vi "HFRR ADV v043.vi"() -> ()   [LabVIEW 2025] (continued)
            "LVDT MIN" <- w2050
            "LVDT MAX" <- w2049
            "LVDT Peak" <- w2048
            "pizo raw" <- w2047
            "cof" <- w2045
            "Frictioin Force Raw" <- w2046
          }
        }
      }
      frame Error {
      }
    }
    n1779 = local read "Quit"() -> (w1964:bool)
  }
  n1780 = disable-structure shown="Disabled" {
    disable-tunnel: errorcluster {"status"=TRUE, "code"=0, "source"="Init"} ("error IO") -> [w2109 _]
    disable-tunnel: [w2107 _] -> w49
    frame Disabled {
      n1781 = while {
        shift-right: [w2125] -> w2111
        shift-left: _ -> [w2116]
        shift-right: [w2124] -> w2110
        shift-left: w2109 -> [w2118]
        tunnel: [w2113] -> w2107
        tunnel: [w2123] -> _
        i -> [w2123]
        stop <- w2113 stop-if-true
        n1782 = local read "Port 1a"() -> (w2119:bool)
        n1783 = local read "Port 3"() -> (w2120:bool)
        n1784 = local read "Com Port 1"() -> (w2117:refnum<visa-resource-name>)
        n1785 = Or(x=w2120, y=w2119) -> (x .or. y?=w2122:bool)
        n1786 = Unbundle(w2118) -> ("status"=→"Port 3":bool)  [unwired: 2 out]
        n1787 = Not Equal?(x=w2117, y=w2116) -> (x != y?=w2114:bool)
        n1788 = case shown="True" w2122 {
          frame False {
            w2128 = TRUE ("Visible")
            n1789 = property on="Port 1a" class="Bool (strict)"("Visible"=w2128) -> ()  [unwired: 2 in, 2 out]
            n1790 = property on="Port 3" class="Bool (strict)"("Visible"=w2128) -> ()  [unwired: 2 in, 2 out]
          }
          frame True {
            w2129 = TRUE ("Visible")
            n1791 = property on="Port 1a" class="Bool (strict)"("Visible"=w2129) -> ()  [unwired: 2 in, 2 out]
            n1792 = property on="Port 3" class="Bool (strict)"("Visible"=w2129) -> ()  [unwired: 2 in, 2 out]
          }
        }
        n1793 = Wait (ms)(milliseconds to wait=u32 40) -> ()  [unwired: 1 out]
        n1794 = case shown="True" w2114 {
          tunnel: [w2126 errorcluster {"status"=TRUE, "code"=0, "source"="Init"} ("error out")] -> w2115
          tunnel: w2118 -> [w2126 _]
          frame False {
          }
          frame True {
          }
        }
        n1795 = case shown="Error" w2115 {
          selector: w2115 -> [w2136 w2154]
          tunnel: [w2139 w2158] -> w2125
          tunnel: [w2138 w2152] -> w2124
          tunnel: w2116 -> [w2137 w2156]
          frame No Error {
            n1796 = property class="Instr"(reference=w2137, error in=w2136) -> (reference out=w2134:refnum<visa-resource-name>, error out=w2135:errorcluster, "Serial Settings:Number of Bytes at Serial Port"=w2131:u32)
            n1797 = Greater?(x=w2131, y=u32 5) -> (0:w2130:bool)
            n1798 = Not(x=w2130) -> (.not. x?=→"Port 1a":bool)
            n1799 = while {
              tunnel: [w2147] -> w2138
              tunnel: [w2146] -> w2139
              tunnel: w2135 -> [w2145]
              tunnel: w2134 -> [w2144]
              stop <- TRUE stop-if-true
              n1800 = property class="Instr" props=["Serial Settings:Number of Bytes at Serial Port"](reference=w2144, error in=w2145) -> (reference out=w2149:refnum<visa-resource-name>, error out=w2148:errorcluster)  [unwired: 1 out]
              n1801 = VISA Read(VISA resource name=w2149, byte count=u32 50, error in (no error)=w2148) -> (VISA resource name out=w2146:refnum<visa-resource-name>, read buffer=w2141:string, error out=w2147:errorcluster)  [unwired: 1 out]
              n1802 = Wait (ms)(milliseconds to wait=u32 5) -> ()  [unwired: 1 out]
            }
          }
          frame Error {
            w2164 = u16 0 items=["None", "XON/XOFF", "RTS/CTS", "XON/XOFF & RTS/CTS", "DTR/DSR", "XON/XOFF & DTR/DSR"] ("flow control (0:none)  2")
            w2162 = u16 10 items=["1.0"=10, "1.5"=15, "2.0"=20] ("stop bits 2")
            w2160 = u16 0 items=["None", "Odd", "Even", "Mark", "Space"] ("parity 2")
            w2161 = u32 10000  # timeout (10sec)
            n1803 = VISA Close(VISA resource name=w2156, error in (no error)=w2154) -> (error out=w2157:errorcluster)
            n1804 = local write "Port 1a"(FALSE ("Port 1a")) -> ()
            n1805 = local read "Com Port 1"() -> (w2151:refnum<visa-resource-name>)
            n1806 = call <vilib>:"Clear Errors.vi"("error in (no error)"=w2157) -> ("error out"=w2155:errorcluster)  [unwired: 5 in, 1 out]
            n1807 = call-poly "VISA Configure Serial Port"("VISA resource name"=w2151, "timeout (10sec)"=w2161, "baud rate (9600)"=u32 250000 ("baud rate  2"), "data bits (8)"=u16 8 ("data bits  2"), "parity (0:none)"=w2160, "error in (no error)"=w2155, "stop bits (10: 1 bit)"=w2162, "flow control (0:none)"=w2164) -> ("VISA resource name out"=w2165:refnum<visa-resource-name>, "error out"=w2166:errorcluster)  [unwired: 6 in]
            n1808 = flat-sequence {
              tunnel: w2165 -> [w2168]
              tunnel: w2166 -> [w2167]
              tunnel: [w2168] -> w2158
              tunnel: [w2167] -> w2152
              frame #0 {
                n1809 = Wait (ms)(milliseconds to wait=u32 50) -> ()  [unwired: 1 out]
              }
            }
            "Residual Uno" <- ""
          }
        }
        n1810 = local read "Quit"() -> (w2113:bool)
        "Error Uno" <- w2118
      }
      n1811 = VISA Close(VISA resource name=w2111, error in (no error)=w2110) -> (error out=w2108:errorcluster)
      n1812 = call <vilib>:"Clear Errors.vi"("error in (no error)"=w2108) -> ()  [unwired: 5 in, 2 out]
    }
    frame Enabled {
    }
  }
  n1813 = while {
    stop <- w2179 stop-if-true
    # "V0OLTAGE TO STROKE (peice vise calibration)"
    n1814 = local read "LVDT MIN"() -> (w2171:dbl)
    n1815 = local read "LVDT Peak"() -> (w2170:dbl)
    n1816 = Wait (ms)(milliseconds to wait=u32 10) -> ()  [unwired: 1 out]
    n1817 = formula code="// Dynamic Parameterized Linear Interpolation Node\n// Inputs: vpp_val, voltages (Array), distances (Array)\n// Outputs: stroke\n\nint i = 0;\nint segments = 11; // 12 points make 11 interpolation segments\n\n// 1. Lower Boundary Clamp\nif (vpp_val <= voltages[0]) {\n    stroke = distances[0];\n}\n// 2. Upper Boundary Clamp\nelse if (vpp_val >= voltages[segments]) {\n    stroke = distances[segments];\n}\n// 3. Dynamic Segment Search Loop\nelse {\n    stroke = distances[0]; // Fallback baseline\n    for (i = 0; i < segments; i++) {\n        if (vpp_val >= voltages[i] && vpp_val <= voltages[i+1]) {\n            // Standard linear interpolation formula using array lookups\n            stroke = distances[i] + (vpp_val - voltages[i]) * (distances[i+1] - distances[i]) / (voltages[i+1] - voltages[i]);\n            break; // Segment found, safely exit the loop\n        }\n    }\n}"("vpp_val"=w2170, "voltages"="calibration values", "distances"="STROKE") -> ("stroke"=→"LVDT STROKE":dbl)
    n1818 = local read "Calibration Tare Value"() -> (w2175:dbl)
    n1819 = local read "Calibration Tare"() -> (w2173:bool)
    n1820 = Subtract(x=w2171, y=w2175) -> (x-y=→"LVDT STROKE  Calibration":dbl)
    n1821 = case shown="True" w2173 {
      selector: w2173 -> [_ w2181]
      tunnel: w2171 -> [_ w2182]
      frame False {
      }
      frame True {
        n1822 = Not(x=w2181) -> (.not. x?=w2180:bool)
        n1823 = local write "Calibration Tare"(w2180) -> ()
        "Calibration Tare Value" <- w2182
      }
    }
    n1824 = local read "Quit"() -> (w2179:bool)
  }
  n1825 = while {
    stop <- w2205 stop-if-true
    n1826 = local read "Due read"() -> (w2203:string)
    n1827 = call <vilib>:"High Resolution Polling Wait.vi"("seconds to wait"=0.02) -> ()  [unwired: 10 in, 1 out]
    n1828 = local read "Frictioin Force Raw"() -> (w2185:dbl)
    n1829 = Spreadsheet String To Array(delimiter (Tab)=";", format string="", spreadsheet string=w2203, array type (2D Dbl)=string[] []) -> (array=w2200:string[])
    n1830 = Fract/Exp String To Number(string=w2200) -> (number=w2199:dbl[])  [unwired: 3 in, 1 out]
    n1831 = call <vilib>:"Median Filter PtByPt.vi"("rank"=2, "x"=w2185) -> ("Filtered x"=→"Friction":dbl)  [unwired: 2 in, 1 out]
    n1832 = Index Array(array=w2199) -> (element #1=→"Sample Temperature 2":dbl, element #2=→"Target Sample Temperature":dbl, element #3=→"Current Duty Cycle":dbl, element #4=→"Ambient Temperature":dbl, element #5=→"Dac Status":dbl, element #6=→"Vpp":dbl, element #7=→"Active Error Code":dbl, element #8=→"Kp":dbl, element #9=→"Ki":dbl, element #10=→"Kd":dbl, element #11=→"SampleRaw":dbl, element #12=→"AmbRaw":dbl)  [unwired: 12 in]
    n1833 = local read "Quit"() -> (w2205:bool)
  }
  n1834 = while {
    shift-right: [w2219] -> w45
    shift-left: _ -> [w2211]
    shift-right: [w2206] -> w44
    shift-left: errorcluster {"status"=FALSE, "code"=0, "source"="Init"} ("error out") -> [w2213]
    tunnel: [w2208] -> w48
    tunnel: [w2218] -> _
    i -> [w2218]
    stop <- w2208 stop-if-true
    n1835 = local read "Com Port 2"() -> (w2212:refnum<visa-resource-name>)
    n1836 = local read "Port 2a"() -> (w2214:bool)
    n1837 = Unbundle(w2213) -> ("status"=→"Port 4":bool)  [unwired: 2 out]
    n1838 = call <vilib>:"High Resolution Polling Wait.vi"("seconds to wait"=0.02) -> ()  [unwired: 10 in, 1 out]
    n1839 = local read "Port 4"() -> (w2215:bool)
    n1840 = Not Equal?(x=w2212, y=w2211) -> (x != y?=w2210:bool)
    n1841 = Or(x=w2215, y=w2214) -> (x .or. y?=w2217:bool)
    n1842 = case shown="False" w2217 {
      frame False {
        w2222 = TRUE ("Visible")
        n1843 = property on="Port 2a" class="Bool (strict)"("Visible"=w2222) -> ()  [unwired: 2 in, 2 out]
        n1844 = property on="Port 4" class="Bool (strict)"("Visible"=w2222) -> ()  [unwired: 2 in, 2 out]
      }
      frame True {
        w2223 = TRUE ("Visible")
        n1845 = property on="Port 2a" class="Bool (strict)"("Visible"=w2223) -> ()  [unwired: 2 in, 2 out]
        n1846 = property on="Port 4" class="Bool (strict)"("Visible"=w2223) -> ()  [unwired: 2 in, 2 out]
      }
    }
    n1847 = case shown="True" w2210 {
      tunnel: [w2220 errorcluster {"status"=TRUE, "code"=0, "source"="Init"} ("error out")] -> w2209
      tunnel: w2213 -> [w2220 _]
      frame False {
      }
      frame True {
      }
    }
    n1848 = case shown="No Error" w2209 {
      selector: w2209 -> [w2236 w2267]
      tunnel: [w2229 w2272] -> w2219
      tunnel: [w2237 w2265] -> w2206
      tunnel: w2211 -> [w2238 w2270]
      frame No Error {
        n1849 = property class="Instr" props=["Serial Settings:Number of Bytes at Serial Port"](reference=w2238, error in=w2236) -> (reference out=w2230:refnum<visa-resource-name>, error out=w2235:errorcluster)  [unwired: 1 out]
        n1850 = while {
          tunnel: [w2246] -> w2231
          tunnel: [w2245] -> w2232
          tunnel: w2235 -> [w2244]
          tunnel: w2230 -> [w2243]
          tunnel: [w2242] -> _
          i -> [w2242]
          stop <- TRUE stop-if-true
          n1851 = property class="Instr" props=["Serial Settings:Number of Bytes at Serial Port"](reference=w2243, error in=w2244) -> (reference out=w2248:refnum<visa-resource-name>, error out=w2247:errorcluster)  [unwired: 1 out]
          n1852 = VISA Read(VISA resource name=w2248, byte count=u32 1000, error in (no error)=w2247) -> (VISA resource name out=w2245:refnum<visa-resource-name>, read buffer=→"Due read":string, error out=w2246:errorcluster)  [unwired: 1 out]
        }
        n1853 = local read "Due Write"() -> (w2228:string)
        n1854 = call <vilib>:"Trim Whitespace.vi"("string"=w2228) -> ("trimmed string"=w2227:string)  [unwired: 1 in]
        n1855 = Not Equal?(x=w2227, y="") -> (x != y?=w2233:bool)
        n1856 = VISA Flush I/O Buffer(VISA resource name=w2232) -> (VISA resource name out=w2225:refnum<visa-resource-name>, error out=→"error out 10":errorcluster)  [unwired: 2 in]
        n1857 = case shown="True" w2233 {
          tunnel: w2225 -> [w2250 w2255]
          tunnel: [w2250 w2259] -> w2229
          tunnel: w2231 -> [w2249 w2254]
          tunnel: [w2249 w2257] -> w2237
          tunnel: w2227 -> [_ w2253]
          tunnel: [_ w2256] -> _
          frame False {
            # "DATA  WRITE LOOP"
          }
          frame True {
            n1858 = Concatenate Strings(w2253, "\r\n") -> (w2252:string)
            n1859 = VISA Write(VISA resource name=w2255, write buffer=w2252, error in (no error)=w2254) -> (VISA resource name out=w2259:refnum<visa-resource-name>, return count=w2256:u32, error out=w2258:errorcluster)
            n1860 = flat-sequence {
              tunnel: w2258 -> [w2261]
              tunnel: [w2261] -> w2257
              frame #0 {
                n1861 = local write "Due Write"("" ("Command")) -> ()
                n1862 = Wait (ms)(milliseconds to wait=u32 5) -> ()  [unwired: 1 out]
              }
            }
          }
        }
        "Port 2a" <- TRUE ("Port 2a")
      }
      frame Error {
        w2278 = u16 0 items=["None", "XON/XOFF", "RTS/CTS", "XON/XOFF & RTS/CTS", "DTR/DSR", "XON/XOFF & DTR/DSR"] ("flow control (0:none)  2")
        w2276 = u16 10 items=["1.0"=10, "1.5"=15, "2.0"=20] ("stop bits 2")
        w2274 = u16 0 items=["None", "Odd", "Even", "Mark", "Space"] ("parity 2")
        w2275 = u32 10000  # timeout (10sec)
        n1863 = VISA Clear(VISA resource name=w2270, error in (no error)=w2267) -> (VISA resource name out=w2269:refnum<visa-resource-name>, error out=w2268:errorcluster)
        n1864 = VISA Close(VISA resource name=w2269, error in (no error)=w2268) -> (error out=w2271:errorcluster)
        n1865 = call <vilib>:"Clear Errors.vi"("error in (no error)"=w2271) -> ()  [unwired: 5 in, 2 out]
        n1866 = local write "Port 2a"(FALSE ("Port 2a")) -> ()
        n1867 = local read "Com Port 2"() -> (w2264:refnum<visa-resource-name>)
        "visa due" <- w2264
        n1868 = call-poly "VISA Configure Serial Port"("VISA resource name"=w2264, "timeout (10sec)"=w2275, "baud rate (9600)"=u32 250000 ("baud rate  2"), "data bits (8)"=u16 8 ("data bits  2"), "parity (0:none)"=w2274, "stop bits (10: 1 bit)"=w2276, "flow control (0:none)"=w2278) -> ("VISA resource name out"=w2279:refnum<visa-resource-name>, "error out"=w2280:errorcluster)  [unwired: 7 in]
        n1869 = flat-sequence {
          tunnel: w2279 -> [w2282]
          tunnel: w2280 -> [w2281]
          tunnel: [w2282] -> w2272
          tunnel: [w2281] -> w2265
          frame #0 {
            n1870 = Wait (ms)(milliseconds to wait=u32 50) -> ()  [unwired: 1 out]
          }
        }
        "Residual Due" <- ""
      }
    }
    "error out 9" <- w2206
    n1871 = local read "Quit"() -> (w2208:bool)
    "Error Due" <- w2213
  }
  n1872 = local write "FRICVALZ"(0.0 ("FRICVALZ")) -> ()
  n1873 = property on="RUN" class="Bool (strict)"("Visible"=TRUE) -> ()  [unwired: 2 in, 2 out]
  n1874 = while {
    tunnel: [w2297] -> _
    tunnel: [w2284] -> w58
    i -> [w2297]
    stop <- w2284 stop-if-true
    n1875 = local read "conststatus"() -> (w2288:dbl)
    n1876 = local read "Main Tab"() -> (w2286:T2)
    n1877 = local read "EDIT"() -> (w2303:bool)
    n1878 = local read "Rate"() -> (w2302:dbl)
    n1879 = case shown="True" w2303 {
      tunnel: [FALSE TRUE] -> _
      frame False {
      }
      frame True {
      }
    }
    n1880 = Equal?(x=w2286, y=T28."About" ("Main Tab")) -> (x = y?=w2295:bool)
    n1881 = Equal?(x=w2288, y=0.0) -> (x = y?=w2289:bool)
    n1882 = Divide(x=1.0, y=w2302) -> (x/y=w2298:dbl)
    "Time 2" <- w2298
    n1883 = case shown="True" w2289 {
      frame False {
      }
      frame True {
        # "C:\\WinDucom\\calibrate WO 2391.dcf"
        n1884 = local write "Lan flag"(22) -> ()
        n1885 = local write "conststatus"(10.0 ("rpm value : 2")) -> ()
        n1886 = String To Path(string="C:\\LAB-IQ\\calibrate WO 2465.dcf") -> (path=w2309:path)
        n1887 = Open/Create/Replace File "Open File"(file path (use dialog)=w2309) -> (refnum out=w2307:refnum<file>)  [unwired: 5 in, 2 out]
        n1888 = for {
          N: 23 -> [_]
          tunnel: w2307 -> [w2318]
          i -> [w2312]
          (unwired) TRUE ("line mode (F)")
          n1889 = Read from Text File "Read File"(file (use dialog)=w2318) -> (text=w2317:string)  [unwired: 3 in, 3 out]
          n1890 = Match Pattern(string=w2317, regular expression="]") -> (after substring=w2315:string)  [unwired: 1 in, 3 out]
          n1891 = String Subset(string=w2317, offset (0)=5, length (rest)=10 ("length (rest)")) -> (substring=w2310:string)
          n1892 = Fract/Exp String To Number(string=w2310) -> (number=w2311:dbl)  [unwired: 3 in, 1 out]
          n1893 = Match Pattern(string=w2315, regular expression="-") -> (before substring=w2313:string)  [unwired: 1 in, 3 out]
          n1894 = case shown="10" w2312 {
            tunnel: w2311 -> [_ _ _ _ _ _ _ _ _ _ w2325 _ _ _ _ _ _ _ _ _ _ _ _ _]
            tunnel: w2313 -> [_ _ _ _ w2321 w2322 w2323 _ _ _ _ _ _ _ _ _ _ _ _ _ w2326 w2327 w2328 _]
            frame 0 {
            }
            frame 1 {
            }
            frame 2 {
            }
            frame 3 {
            }
            frame 4 {
              n1895 = local write "Com Port 1"(w2321) -> ()
            }
            frame 5 {
              n1896 = local write "Com Port 2"(w2322) -> ()
              n1897 = local write "visa due"(w2322) -> ()
            }
            frame 6 {
              n1898 = String To Path(string=w2323) -> (path=w2324:path)
              n1899 = local write "File Path"(w2324) -> ()
              "String" <- w2323
            }
            frame 7 {
            }
            frame 8 {
            }
            frame 9 {
            }
            frame 10 {
              n1900 = local write "Language Selection"(w2325) -> ()
            }
            frame 11 {
            }
            frame 12 {
            }
            frame 13 {
            }
            frame 14 {
            }
            frame 15 {
            }
            frame 16 {
            }
            frame 17 {
            }
            frame 18 {
            }
            frame 21 {
            }
            frame 22 {
              n1901 = local write "Com Port 3"(w2326) -> ()
            }
            frame 20 {
              n1902 = local write "Camera Port :"(w2327) -> ()
            }
            frame 19 {
              n1903 = local write "C3 :"(w2328) -> ()
            }
            frame 23, Default {
            }
          }
        }
      }
    }
    n1904 = Select(t=u32 2500 ("milliseconds to wait"), s=w2295, f=u32 500 ("milliseconds to wait")) -> (s? t:f=w2293:u32)
    n1905 = Multiply(x=w2298, y=w2293) -> (x*y=w2300:dbl)
    n1906 = call "Elapsed Time2"("Time Target (s)"=w2300, "Auto Reset"=TRUE) -> ("Time has Elapsed"=w2290:bool)  [unwired: 10 in, 7 out]
    n1907 = case shown="True" w2290 {
      frame False {
      }
      frame True {
        n1908 = stacked-sequence {
          frame #0 {
            # "DATA PROCESSING"
            # "115 mV/N"
            n1909 = local read "Sample Temperature 2"() -> (w2331:dbl)
            n1910 = local read "RH Numeric:"() -> (→"Humidity ( %RH )":dbl)
            n1911 = local read "FRICVALZ"() -> (w2348:dbl)
            n1912 = local read "Friction"() -> (w2334:dbl)
            n1913 = call <vilib>:"Mean PtByPt.vi"("x"=w2331, "sample length"=100) -> ("mean"=w2330:dbl)  [unwired: 2 in, 1 out]
            "TEMP 2" <- w2330
            "TEMP 3" <- w2330
            n1914 = Subtract(x=w2334, y=w2348) -> (x-y=w2343:dbl)
            "FF 2" <- w2343
            "FF 4" <- w2343
            n1915 = local read "Ambient Temperature"() -> (→"AIR TEMP":dbl)
            n1916 = local read "TEMP"() -> (w2347:dbl)
            n1917 = local write "FF 3"(w2343) -> ()
            n1918 = Compound Arithmetic op=OR("FRICVALZ 4", "FRICVALZ 3", "FRICVALZ 2") -> (w2339:bool)
            n1919 = case shown="True" w2339 {
              tunnel: w2334 -> [_ w2354]
              frame False {
              }
              frame True {
                w2353 = FALSE ("FRICVALZ")
                n1920 = local write "FRICVALZ 3"(w2353) -> ()
                n1921 = local write "FRICVALZ 2"(w2353) -> ()
                n1922 = local write "FRICVALZ 4"(w2353) -> ()
                "FRICVALZ" <- w2354
              }
            }
            n1923 = Not A Number/Path/Refnum?(number/path/refnum=w2347) -> (NaN/Path/Refnum?=w2346:bool)
            n1924 = Not A Number/Path/Refnum?(number/path/refnum=w2343) -> (NaN/Path/Refnum?=w2345:bool)
            n1925 = Divide(x=w2343, y=1.96) -> (x/y=w2340:dbl)
            n1926 = Compound Arithmetic op=OR(w2346, w2345) -> (w2344:bool)
            n1927 = Not A Number/Path/Refnum?(number/path/refnum=w2340) -> (NaN/Path/Refnum?=w2341:bool)
            n1928 = case shown="True" w2344 {
              frame False {
              }
              frame True {
                n1929 = local write "TEMP"(0.0 ("TEMP")) -> ()
                n1930 = local write "FF 2"(0.0 ("FF 2")) -> ()
                n1931 = local write "reinit"(TRUE ("reinit")) -> ()
              }
            }
            n1932 = local write "TEMP"(w2330) -> ()
            n1933 = Select(t=0.0, s=w2341, f=w2340) -> (s? t:f=w2333:dbl)
            "COF 2" <- w2333
            n1934 = local write "COF 3"(w2333) -> ()
          }
        }
      }
    }
    n1935 = Wait (ms)(milliseconds to wait=u32 50) -> ()  [unwired: 1 out]
    n1936 = local read "Quit"() -> (w2284:bool)
    "Rate" <- 2500.0 ("No of Samples")
  }
  n1937 = while {
    tunnel: [w2374] -> _
    tunnel: [w2357] -> w60
    tunnel: w5 -> [_]
    i -> [w2374]
    stop <- w2357 stop-if-true
    # "C:\\LAB-IQ-NXT\\Scar View.exe"
    n1938 = local read "OK Button 16"() -> (w2364:bool)
    n1939 = local read "Main Tab"() -> (w2358:T2)
    n1940 = local read "service 3"() -> (w2359:bool)
    n1941 = local read "OPEN 6"() -> (w2361:bool)
    n1942 = local read "EDIT 2"() -> (w2363:bool)
    n1943 = flat-sequence {
      frame #0 {
        n1944 = stacked-sequence {
          frame #0 {
            n1945 = local read "EDIT"() -> (w2852:bool)
            n1946 = case shown="False" w2852 {
              tunnel: [u8 2 ("Disabled") u8 0 ("Disabled")] -> _
              frame False {
                w2854 = FALSE
                n1947 = local write "Password"("") -> ()
                n1948 = local write "x = y?"(w2854) -> ()
                n1949 = property on="Password" class="Str"("Visible"=w2854) -> ()  [unwired: 2 in, 2 out]
              }
              frame True {
                n1950 = property on="Password" class="Str"("Visible"=TRUE) -> ()  [unwired: 2 in, 2 out]
              }
            }
            "dipl pwd" <- "@143$\n" ("dipl pwd")
          }
          frame #1 {
          }
          frame #2 {
          }
          frame #3 {
          }
          frame #4 {
            n1951 = String To Byte Array(string="Password") -> (unsigned byte array=w2865:u8[])
            n1952 = Search 1D Array(1D array=w2865, element=u8 10) -> (index of element=w2863:i32)  [unwired: 1 in]
            n1953 = Index Array(array=w2865, index=w2863) -> (element=w2864:u8)
            n1954 = Equal?(x=w2864, y=10) -> (x = y?=w2860:bool)
            n1955 = case shown="True" w2860 {
              frame False {
              }
              frame True {
                # "password"
                # "password"
                n1956 = local read "Password"() -> (w2877:string)
                n1957 = String To Byte Array(string=w2877) -> (unsigned byte array=w2880:u8[])
                n1958 = String To Byte Array(string="@143$\n") -> (unsigned byte array=w2867:u8[])
                n1959 = Array Size(array=w2880) -> (size(s)=w2876:i32)
                n1960 = Array Size(array=w2867) -> (size(s)=w2872:i32)
                n1961 = for {
                  N: w2876 -> [_]
                  tunnel: w2880 -> [w2893]
                  tunnel: [w2891] -> w2881 mode=indexing
                  tunnel: w2876 -> [w2888]
                  i -> [w2889]
                  n1962 = Decrement(x=w2888) -> (x-1=w2887:i32)
                  n1963 = Index Array(array=w2893, index=w2889) -> (element=w2892:u8)
                  n1964 = Equal?(x=w2889, y=w2887) -> (x = y?=w2886:bool)
                  n1965 = Number To Decimal String(number=w2892) -> (decimal integer string=w2890:string)  [unwired: 1 in]
                  n1966 = Select(t="", s=w2886, f="\r") -> (s? t:f=w2883:string)
                  n1967 = Concatenate Strings(w2890, w2883) -> (w2891:string)
                }
                n1968 = for {
                  N: w2872 -> [_]
                  tunnel: w2867 -> [w2904]
                  tunnel: [w2902] -> w2870 mode=indexing
                  tunnel: w2872 -> [w2899]
                  i -> [w2900]
                  n1969 = Decrement(x=w2899) -> (x-1=w2898:i32)
                  n1970 = Index Array(array=w2904, index=w2900) -> (element=w2903:u8)
                  n1971 = Equal?(x=w2900, y=w2898) -> (x = y?=w2897:bool)
                  n1972 = Number To Decimal String(number=w2903) -> (decimal integer string=w2901:string)  [unwired: 1 in]
                  n1973 = Select(t="", s=w2897, f="\r") -> (s? t:f=w2894:string)
                  n1974 = Concatenate Strings(w2901, w2894) -> (w2902:string)
                }
                n1975 = local read "file path"() -> (w2866:path)
                n1976 = call <vilib>:"Read Characters From File.vi"("file path (dialog if empty)"=w2866) -> ("character string"=w2879:string)  [unwired: 5 in, 3 out]
                "string" <- w2879
                n1977 = flat-sequence {
                  tunnel: [w2882] -> _
                  frame #0 {
                    w2882 = ""
                    n1978 = local write "Password"(w2882) -> ()
                  }
                }
                n1979 = Concatenate Strings(w2870) -> (w2871:string)
                n1980 = Concatenate Strings(w2879) -> (w2878:string)
                n1981 = Concatenate Strings(w2881) -> (w2874:string)
                n1982 = Equal?(x=w2874, y=w2878) -> (x = y?=w2869:bool)
                n1983 = Equal?(x=w2874, y=w2871) -> (x = y?=w2875:bool)
                n1984 = Or(x=w2869, y=w2875) -> (x .or. y?=→"x = y?":bool)
              }
            }
          }
        }
        n1985 = local read "x = y?"() -> (w2850:bool)
        n1986 = And(x="EDIT", y=w2850) -> (x .and. y?=w2848:bool)
        n1987 = case shown="True" w2848 {
          tunnel: [u8 2 ("Disabled") u8 0 ("Disabled")] -> w2847
          tunnel: [w3054 TRUE ("Visible")] -> w2846
          frame False {
            w3054 = FALSE ("Visible")
            n1988 = local write "EDIT 2"(w3054) -> ()
          }
          frame True {
          }
        }
        n1989 = case shown="True" "SAVE" {
          frame False {
          }
          frame True {
            n1990 = stacked-sequence {
              seq-local: [w2909 _ _] -> [_ w3050 _]
              frame #0 {
                w2905 = 0.0 ("number")
                w2906 = 0.0 ("number")
                (unwired) i16 5 ("precision (6)")
                # "[CH1]    - FF\n[CH2]   - TEMPERATURE\n[CH3]    - Humidity\n[CH4]    - AIR TEMP\n[CH5]\\- Visa Uno\n[CH6] \\- Visa Due\n[CH7]  \\- file path\n[CH8]   - Displacement Gain\n[CHA]   - Stroke Gain\n[CHB]   - Stroke PID Gain\n[CHC]   -Language Selection\n[CHD]   -Power +\n[CHE]   -Power_\n[CHF]   -Heater\n[CHG]   -Humidity Wet\n[CHH]   -Humidity Dry\n[CHI]   -Integral Time"
                n1991 = local read "Language Selection"() -> (w2952:enum16{"English", "Russian"})
                n1992 = Path To String(path="File Path") -> (string=w2968:string)
                n1993 = Number To Fractional String(number=w2905, width (-)=i16 10 ("precision (6)"), precision (6)=i16 5) -> (F-format string=w2959:string)  [unwired: 1 in]
                n1994 = Number To Fractional String(number=w2952, width (-)=i16 10 ("precision (6)"), precision (6)=i16 5) -> (F-format string=w2948:string)  [unwired: 1 in]
                n1995 = Number To Fractional String(number=w2906, width (-)=i16 10 ("precision (6)"), precision (6)=i16 5) -> (F-format string=w2942:string)  [unwired: 1 in]
                n1996 = Number To Fractional String(number=w2906, width (-)=i16 10 ("precision (6)"), precision (6)=i16 5) -> (F-format string=w2939:string)  [unwired: 1 in]
                n1997 = Number To Fractional String(number=w2906, width (-)=i16 10 ("precision (6)"), precision (6)=i16 5) -> (F-format string=w2934:string)  [unwired: 1 in]
                n1998 = Number To Fractional String(number=w2906, width (-)=i16 10 ("precision (6)"), precision (6)=i16 5) -> (F-format string=w2931:string)  [unwired: 1 in]
                n1999 = Number To Fractional String(number=w2906, width (-)=i16 10 ("precision (6)"), precision (6)=i16 5) -> (F-format string=w2926:string)  [unwired: 1 in]
                n2000 = local read "Com Port 1"() -> (w2908:refnum<visa-resource-name>)
                n2001 = local read "Com Port 2"() -> (w2907:refnum<visa-resource-name>)
                n2002 = Concatenate Strings(w2968, "\\" ("string")) -> (w2967:string)
                n2003 = Number To Fractional String(number=w2905, width (-)=i16 10 ("precision (6)"), precision (6)=i16 5) -> (F-format string=w3000:string)  [unwired: 1 in]
                n2004 = Number To Fractional String(number=w2905, width (-)=i16 10 ("precision (6)"), precision (6)=i16 5) -> (F-format string=w2999:string)  [unwired: 1 in]
                n2005 = Number To Fractional String(number=w2905, width (-)=i16 10 ("precision (6)"), precision (6)=i16 5) -> (F-format string=w2993:string)  [unwired: 1 in]
                n2006 = Number To Fractional String(number=w2905, width (-)=i16 10 ("precision (6)"), precision (6)=i16 5) -> (F-format string=w2987:string)  [unwired: 1 in]
                n2007 = Number To Fractional String(number=w2905, width (-)=i16 10 ("precision (6)"), precision (6)=i16 5) -> (F-format string=w2960:string)  [unwired: 1 in]
                n2008 = Concatenate Strings("[CHA]" ("string"), w2959, "- Stroke Gain" ("string"), "\r") -> (w2953:string)
                n2009 = Concatenate Strings("[CHC]" ("string"), w2948, "-Language Selection" ("string"), "\r") -> (w2945:string)
                n2010 = Concatenate Strings("[CHD]" ("string"), w2942, "-Power +" ("string"), "\r") -> (w2924:string)
                n2011 = Concatenate Strings("[CHG]" ("string"), w2931, "-Humidity Wet" ("string"), "\r") -> (w2921:string)
                n2012 = Concatenate Strings("[CHH]" ("string"), w2926, "-Humidity Dry" ("string"), "\r") -> (w2920:string)
                n2013 = Concatenate Strings("[CH1]" ("string"), w3000, " - FF" ("string"), "\r") -> (w2998:string)
                n2014 = Concatenate Strings("[CH2]" ("string"), w2999, " - TEMPERATURE" ("string"), "\r") -> (w2997:string)
                n2015 = Concatenate Strings("[CH3]" ("string"), w2993, " - Humidity" ("string"), "\r") -> (w2990:string)
                n2016 = Concatenate Strings("[CH4]" ("string"), w2987, " - AIR TEMP" ("string"), "\r") -> (w2983:string)
                n2017 = Concatenate Strings("[CH5]" ("string"), w2908, "- Visa Uno" ("string"), "\r") -> (w2976:string)
                n2018 = Concatenate Strings("[CH6]" ("string"), w2907, "- Visa Due" ("string"), "\r") -> (w2971:string)
                n2019 = Concatenate Strings("[CH7]" ("string"), w2967, "- file path" ("string"), "\r") -> (w2970:string)
                n2020 = Concatenate Strings("[CH8]" ("string"), w2960, "- Displacement Gain" ("string"), "\r") -> (w2963:string)
                n2021 = Concatenate Strings("[CHE]" ("string"), w2939, "-Power_" ("string"), "\r") -> (w2923:string)
                n2022 = Concatenate Strings("[CHF]" ("string"), w2934, "-Heater" ("string"), "\r") -> (w2922:string)
                n2023 = Concatenate Strings(w2998, w2997, w2990, w2983, w2976, w2971, w2970, w2963, w2953, w2945, w2924, w2923, w2922, w2921, w2920) -> (w2909:string)
                "gain" <- w2909
              }
              frame #1 {
                w3011 = 0.0 ("number")
                n2024 = local read "Camera Port :"() -> (w3014:string)
                n2025 = local read "C3 :"() -> (w3022:refnum<visa-resource-name>)
                n2026 = local read "Com Port 3"() -> (w3023:refnum<visa-resource-name>)
                n2027 = Concatenate Strings("[CH8]" ("string"), w3014, "- Visa Camera" ("string"), "\r") -> (w3013:string)
                n2028 = Concatenate Strings("[CH7]" ("string"), w3022, "- Visa Humidity" ("string"), "\r") -> (w3018:string)
                n2029 = Number To Fractional String(number=w3011, width (-)=i16 10 ("precision (6)"), precision (6)=i16 5) -> (F-format string=w3038:string)  [unwired: 1 in]
                n2030 = Concatenate Strings("[CHL]" ("string"), w3023, "- Visa humid" ("string"), "\r") -> (w3026:string)
                n2031 = Number To Fractional String(number=w3011, width (-)=i16 10 ("precision (6)"), precision (6)=i16 5) -> (F-format string=w3045:string)  [unwired: 1 in]
                n2032 = Concatenate Strings("[CHK]" ("string"), w3038, "-TEMP INTERCEPT" ("string"), "\r") -> (w3034:string)
                n2033 = Concatenate Strings("[SNO]" ("string"), "" ("string"), "-" ("string"), "\r") -> (w3031:string)
                n2034 = Concatenate Strings("[CHJ]" ("string"), w3045, "-AIR TEMP INTERCEPT" ("string"), "\r") -> (w3035:string)
                n2035 = String To Path(string="C:\\LAB-IQ\\calibrate WO 2465.dcf") -> (path=w3024:path)
                n2036 = Concatenate Strings(w3050, w3035, w3034, w3031, w3026, w3018, w3013) -> (w3049:string)
                n2037 = call <vilib>:"Write Characters To File.vi"("append to file? (new file:F)"=FALSE, "character string"=w3049, "file path (dialog if empty)"=w3024) -> ()  [unwired: 2 in, 1 out]
              }
              frame #2 {
                n2038 = local write "Lan flag"(0.0 ("Lan flag")) -> ()
                n2039 = local write "conststatus"(0.0 ("rpm value : 2")) -> ()
                n2040 = local write "SAVE"(FALSE ("OK Button 14")) -> ()
              }
            }
          }
        }
        n2041 = property on="EDIT 2" class="Bool (strict)"("Visible"=w2846) -> ()  [unwired: 2 in, 2 out]
        n2042 = property on="SAVE" class="Bool (strict)"("Visible"=w2846) -> ()  [unwired: 2 in, 2 out]
        n2043 = property on="visa due" class="CmbBox"("Disabled"=w2847) -> ()  [unwired: 2 in, 2 out]
        n2044 = property on="File Path" class="Path"("Disabled"=w2847) -> ()  [unwired: 2 in, 2 out]
        n2045 = property on="Language Selection" class="Enum (strict)"("Visible"=w2846) -> ()  [unwired: 2 in, 2 out]
        n2046 = property on="SPEED OUT:" class="DigNum (strict)"("Disabled"=w2847) -> ()  [unwired: 2 in, 2 out]
      }
    }
    n2047 = local read "RUN"() -> (w2373:bool)
    n2048 = local read "RUN"() -> (w2371:bool)
    n2049 = case shown="True" "EDIT 3" {
      frame False {
      }
      frame True {
        n2050 = local write "EDIT 3"(FALSE ("EDIT 3")) -> ()
        n2051 = local write "Main Tab"(T2."About" ("Main Tab")) -> ()
      }
    }
    n2052 = case shown="False" w2373 {
      frame False {
        n2053 = local read "stopT"() -> (w3061:bool)
        n2054 = case shown="True" w3061 {
          frame False {
          }
          frame True {
            n2055 = local write "stopT"(FALSE) -> ()
          }
        }
      }
      frame True {
        "stopT" <- TRUE
      }
    }
    n2056 = case shown="False" w2371 {
      frame False {
      }
      frame True {
      }
    }
    n2057 = case shown="True" w2363 {
      frame False {
        n2058 = property on="Password 2" class="Str"("Visible"=FALSE) -> ()  [unwired: 2 in, 2 out]
        n2059 = local write "Password 2"("" ("Password")) -> ()
      }
      frame True {
        n2060 = property on="Password 2" class="Str"("Visible"=TRUE) -> ()  [unwired: 2 in, 2 out]
        n2061 = Equal?(x="Password 2", y="HFRR1234") -> (x = y?=w2386:bool)
        n2062 = case shown="True" w2386 {
          tunnel: "Password 2" -> [w2389 _]
          frame False {
            n2063 = String Length(string=w2389) -> (length=w2390:i32)
            n2064 = Greater Than 0?(x=w2390) -> (x > 0?=w2388:bool)
            n2065 = case shown="False" w2388 {
              frame False {
                n2066 = property on="Password 2" class="Str"("Caption.Text"="Password (Advance Setting)") -> ()  [unwired: 2 in, 2 out]
              }
              frame True {
                n2067 = property on="Password 2" class="Str"("Caption.Text"="Incorrect Password!") -> ()  [unwired: 2 in, 2 out]
              }
            }
          }
          frame True {
            n2068 = local write "EDIT 2"(FALSE ("EDIT 2")) -> ()
            n2069 = local write "Password 2"("" ("Password")) -> ()
            n2070 = local write "Main Tab"(T2."Advance" ("Main Tab")) -> ()
            n2071 = local write "Main Dashboard Buttons"(T1."Advance" ("Main Dashboard Buttons")) -> ()
          }
        }
      }
    }
    n2072 = case shown="True" "Prog Uno" {
      frame False {
      }
      frame True {
        n2073 = stacked-sequence {
          frame #0 {
            n2074 = Delete(path (use dialog)=path "C:/LAB-IQ-NXT/UNOCOMPILE.bat" ("working directory")) -> ()  [unwired: 4 in, 3 out]
          }
          frame #1 {
            n2075 = local read "Com Port 1"() -> (w2828:refnum<visa-resource-name>)
            n2076 = Concatenate Strings("cmd.exe /c \"mode " ("command line"), w2828, ":1200,n,8,1\"\n" ("command line")) -> (w2833:string)
            n2077 = Concatenate Strings(w2833, "CD\\\nCD WinDucom\navrdude -C avrdude.conf -v -patmega328p -carduino -P" ("command line"), w2828, " -b115200 -D -Uflash:w:UNO_V20.hex:i\n" ("command line"), "\r") -> (w2835:string)
            "STR" <- w2835
            n2078 = call <vilib>:"Write Characters To File.vi"("append to file? (new file:F)"=FALSE, "character string"=w2835, "file path (dialog if empty)"=path "C:/LAB-IQ/UNOCOMPILE.bat" ("working directory")) -> ()  [unwired: 2 in, 1 out]
          }
          frame #2 {
            n2079 = disable-structure shown="Disabled" {
              frame Disabled {
                w2839 = "cmd.exe  /c \"C:\\LAB-IQ-NXT\\UNOCOMPILE.bat\"" ("string")
                n2080 = local write "Prog Uno"(FALSE ("run minimized? (F)")) -> ()
                n2081 = call <vilib>:"System Exec.vi"("expected output size  (4096)"=u32 65535, "run minimized? (F)"=FALSE, "wait until completion? (T)"=TRUE ("run minimized? (F)"), "working directory"=path "C:/LAB-IQ-NXT", "standard input"=w2839, "command line"=w2839) -> ("error out"=w2838:errorcluster, "standard output"=→"String 42":string)  [unwired: 2 in, 2 out]
                "error out 3" <- w2838
                n2082 = flat-sequence {
                  tunnel: w2838 -> [_]
                  frame #0 {
                  }
                }
              }
              frame Enabled {
              }
            }
          }
        }
      }
    }
    n2083 = case shown="\"ISO 12156\"" "TEST STANDARD" {
      frame "ASTM D6079", Default {
        w2808 = 50.0 ("Hz")
        w2809 = 53.0 ("Set Rh")
        w2811 = 1.0 ("Set Strk")
        w2810 = 60.0 ("Set Temp")
        # "astm hide"
        n2084 = local write "NORMAL LOAD"(200.0 ("NORMAL LOAD")) -> ()
        n2085 = local write "Set Strk"(w2811) -> ()
        n2086 = local write "Set Hz"(w2808) -> ()
        n2087 = local write "Set Temp"(w2810) -> ()
        n2088 = local write "Set Rh"(w2809) -> ()
        n2089 = local write "test time"(75.0 ("test time")) -> ()
        n2090 = local write "Set Stroke:"(w2811) -> ()
        n2091 = local write "Set Humidity:"(w2809) -> ()
        n2092 = local write "Set Frequency:"(w2808) -> ()
        n2093 = local write "Set Temperature:"(w2810) -> ()
        "Test Standard" <- "ASTM D6079" ("Test Standard 2")
      }
      frame "ISO 12156" {
        n2094 = local write "Set Strk"(1.0 ("Set Strk")) -> ()
        n2095 = local write "NORMAL LOAD"(200.0 ("NORMAL LOAD")) -> ()
        n2096 = local write "Set Temp"(60.0 ("Set Temp")) -> ()
        n2097 = local write "test time"(75.0 ("test time")) -> ()
        n2098 = local write "Set Hz"(50.0 ("Hz")) -> ()
        n2099 = local write "Set Rh"(53.0 ("Set Rh")) -> ()
      }
      frame "CEC F-096-A-06" {
        n2100 = local write "Set Strk"(1.0 ("Set Strk")) -> ()
        n2101 = local write "NORMAL LOAD"(200.0 ("NORMAL LOAD")) -> ()
        n2102 = local write "Set Temp"(60.0 ("Set Temp")) -> ()
        n2103 = local write "test time"(75.0 ("test time")) -> ()
        n2104 = local write "Set Hz"(50.0 ("Hz")) -> ()
        n2105 = local write "Set Rh"(53.0 ("Set Rh")) -> ()
      }
      frame "Custom" {
      }
    }
    n2106 = Or(x=w2361, y=w2359) -> (x .or. y?=w2360:bool)
    n2107 = case shown="\"About\"" w2358 {
      tunnel: [T28."Acquire" ("Main Tab") T28."Compare Files" ("Main Tab") T28."About" ("Main Tab")] -> w2369
      frame "Acquire", Default {
      }
      frame "Compare Files" {
      }
      frame "About" {
      }
    }
    n2108 = Or(x=w2364, y="OPEN") -> (x .or. y?=w2365:bool)
    n2109 = case shown="True" w2365 {
      tunnel: w2364 -> [_ w2397]
      frame False {
      }
      frame True {
        n2110 = stacked-sequence {
          tunnel: w2397 -> [_ w2464 _ _]
          frame #0 {
            w2413 = "  " ("String 6")
            n2111 = local write "OPEN"(FALSE ("open")) -> ()
            n2112 = local read "string1 2"() -> (w2401:string)
            n2113 = local read "string1 3"() -> (w2400:string)
            n2114 = local read "string1 4"() -> (w2399:string)
            n2115 = property on="OPEN" class="Bool (strict)"("Visible"=FALSE) -> ()  [unwired: 2 in, 2 out]
            n2116 = local write "String 6"(w2413) -> ()
            n2117 = local write "String 7"(w2413) -> ()
            n2118 = local write "String 8"(w2413) -> ()
            n2119 = local write "String 12"(w2413) -> ()
            n2120 = local read "OK Button 16"() -> (w2398:bool)
            n2121 = String To Path(string=w2401) -> (path=w2409:path)
            n2122 = String To Path(string=w2400) -> (path=w2408:path)
            n2123 = String To Path(string=w2399) -> (path=w2407:path)
            n2124 = case shown="True" w2398 {
              tunnel: [w2414 w2415] -> w2402
              frame False {
                n2125 = local read "string1"() -> (w2414:string)
              }
              frame True {
                n2126 = local read "String Indicator 4"() -> (w2415:string)
              }
            }
            n2127 = Open/Create/Replace File "Open File"(file path (use dialog)=w2409) -> (refnum out=w2405:refnum<file>)  [unwired: 5 in, 2 out]
            n2128 = Open/Create/Replace File "Open File"(file path (use dialog)=w2408) -> (refnum out=w2404:refnum<file>)  [unwired: 5 in, 2 out]
            n2129 = Open/Create/Replace File "Open File"(file path (use dialog)=w2407) -> (refnum out=w2403:refnum<file>)  [unwired: 5 in, 2 out]
            n2130 = while {
              tunnel: w2405 -> [w2427]
              i -> [w2423]
              stop <- w2422 continue-if-true
              (unwired) TRUE ("line mode (F)")
              n2131 = Read from Text File "Read File"(file (use dialog)=w2427) -> (text=w2424:string)  [unwired: 3 in, 3 out]
              n2132 = local write "Numeric 11"(w2423) -> ()
              n2133 = String Length(string=w2424) -> (length=w2426:i32)
              n2134 = Greater?(x=w2426, y=1) -> (0:w2422:bool)
            }
            n2135 = while {
              tunnel: w2404 -> [w2433]
              i -> [w2429]
              stop <- w2428 continue-if-true
              (unwired) TRUE ("line mode (F)")
              n2136 = Read from Text File "Read File"(file (use dialog)=w2433) -> (text=w2430:string)  [unwired: 3 in, 3 out]
              n2137 = local write "Numeric 12"(w2429) -> ()
              n2138 = String Length(string=w2430) -> (length=w2432:i32)
              n2139 = Greater?(x=w2432, y=1) -> (0:w2428:bool)
            }
            n2140 = while {
              tunnel: w2403 -> [w2439]
              i -> [w2435]
              stop <- w2434 continue-if-true
              (unwired) TRUE ("line mode (F)")
              n2141 = Read from Text File "Read File"(file (use dialog)=w2439) -> (text=w2436:string)  [unwired: 3 in, 3 out]
              n2142 = local write "Numeric 13"(w2435) -> ()
              n2143 = String Length(string=w2436) -> (length=w2438:i32)
              n2144 = Greater?(x=w2438, y=1) -> (0:w2434:bool)
            }
            n2145 = String To Path(string=w2402) -> (path=w2410:path)
            n2146 = Open/Create/Replace File "Open File"(file path (use dialog)=w2410) -> (refnum out=w2406:refnum<file>)  [unwired: 5 in, 2 out]
            n2147 = while {
              tunnel: w2406 -> [w2421]
              i -> [w2417]
              stop <- w2416 continue-if-true
              (unwired) TRUE ("line mode (F)")
              n2148 = Read from Text File "Read File"(file (use dialog)=w2421) -> (text=w2418:string)  [unwired: 3 in, 3 out]
              n2149 = local write "Numeric 8"(w2417) -> ()
              n2150 = String Length(string=w2418) -> (length=w2420:i32)
              n2151 = Greater?(x=w2420, y=1) -> (0:w2416:bool)
            }
          }
          frame #1 {
            w2591 = FALSE ("ACTUAL   MERGE")
            # "Sample Temp"
            # "ECR"
            # "COF"
            # "Time\nCOF\nFF\nTemp"
            n2152 = case shown="True" w2464 {
              tunnel: [w2611 w2612] -> w2465
              frame False {
                n2153 = local read "string1"() -> (w2611:string)
              }
              frame True {
                n2154 = local read "String Indicator 4"() -> (w2612:string)
              }
            }
            n2155 = local read "string1 3"() -> (w2509:string)
            n2156 = String To Path(string=w2465) -> (path=w2596:path)
            n2157 = String To Path(string=w2509) -> (path=w2607:path)
            n2158 = local read "Numeric 12"() -> (w2593:i32)
            n2159 = local read "Numeric 8"() -> (w2595:i32)
            n2160 = local read "string1 2"() -> (w2510:string)
            n2161 = local read "string1 4"() -> (w2508:string)
            n2162 = Open/Create/Replace File "Open File"(file path (use dialog)=w2596) -> (refnum out=w2610:refnum<file>, error out=w2609:errorcluster)  [unwired: 5 in, 1 out]
            n2163 = Open/Create/Replace File "Open File"(file path (use dialog)=w2607) -> (refnum out=w2603:refnum<file>, error out=w2604:errorcluster)  [unwired: 5 in, 1 out]
            n2164 = for {
              N: w2595 -> [_]
              tunnel: w2610 -> [w2758]
              tunnel: w2609 -> [w2757]
              tunnel: [w2747] -> w2522 mode=indexing
              tunnel: [w2745] -> w2579 mode=indexing
              tunnel: [w2746] -> w2574 mode=indexing
              tunnel: w2591 -> [_]
              tunnel: [w2739] -> w2576 mode=indexing
              tunnel: [w2735] -> w2545 mode=indexing
              tunnel: [w2731] -> w2520 mode=indexing
              tunnel: [w2727] -> w2501 mode=indexing
              tunnel: [w2722] -> w2461 mode=indexing
              (unwired) TRUE ("line mode (F)")
              # "freq"
              # "Stroke"
              # "Time"
              # "CoF"
              # "Humidity"
              # "Temp"
              # "Air Temp"
              # "ECR"
              n2165 = Read from Text File "Read File"(file (use dialog)=w2758, error in=w2757) -> (text=w2723:string)  [unwired: 2 in, 3 out]
              n2166 = local write "String 6"(w2723) -> ()
              n2167 = String Subset(string=w2723, offset (0)=0, length (rest)=14 ("length (rest)")) -> (substring=w2751:string)
              n2168 = String Subset(string=w2723, offset (0)=35, length (rest)=9 ("length (rest)")) -> (substring=w2748:string)
              n2169 = String Subset(string=w2723, offset (0)=15, length (rest)=9 ("length (rest)")) -> (substring=w2754:string)
              n2170 = Fract/Exp String To Number(string=w2751) -> (number=w2747:dbl)  [unwired: 3 in, 1 out]
              n2171 = Fract/Exp String To Number(string=w2748) -> (number=w2746:dbl)  [unwired: 3 in, 1 out]
              n2172 = Fract/Exp String To Number(string=w2754) -> (number=w2745:dbl)  [unwired: 3 in, 1 out]
              n2173 = String Subset(string=w2723, offset (0)=85, length (rest)=9 ("length (rest)")) -> (substring=w2724:string)
              n2174 = String Subset(string=w2723, offset (0)=25, length (rest)=9 ("length (rest)")) -> (substring=w2730:string)
              n2175 = String Subset(string=w2723, offset (0)=55, length (rest)=9 ("length (rest)")) -> (substring=w2732:string)
              n2176 = String Subset(string=w2723, offset (0)=45, length (rest)=9 ("length (rest)")) -> (substring=w2738:string)
              n2177 = String Subset(string=w2723, offset (0)=65, length (rest)=9 ("length (rest)")) -> (substring=w2744:string)
              n2178 = Fract/Exp String To Number(string=w2730) -> (number=w2727:dbl)  [unwired: 3 in, 1 out]
              n2179 = Fract/Exp String To Number(string=w2724) -> (number=w2722:dbl)  [unwired: 3 in, 1 out]
              n2180 = Fract/Exp String To Number(string=w2732) -> (number=w2731:dbl)  [unwired: 3 in, 1 out]
              n2181 = Fract/Exp String To Number(string=w2738) -> (number=w2735:dbl)  [unwired: 3 in, 1 out]
              n2182 = Fract/Exp String To Number(string=w2744) -> (number=w2741:dbl)  [unwired: 3 in, 1 out]
              n2183 = Add(x=w2741, y=0.0) -> (x+y=w2739:dbl)
            }
            n2184 = for {
              N: w2593 -> [_]
              tunnel: w2604 -> [w2684]
              tunnel: w2603 -> [w2683]
              tunnel: [w2673] -> w2562 mode=indexing
              tunnel: [w2671] -> w2560 mode=indexing
              tunnel: [w2672] -> w2556 mode=indexing
              tunnel: w2591 -> [_]
              tunnel: [w2665] -> w2558 mode=indexing
              tunnel: [w2661] -> w2540 mode=indexing
              tunnel: [w2657] -> w2516 mode=indexing
              tunnel: [w2654] -> w2497 mode=indexing
              tunnel: [w2650] -> w2456 mode=indexing
              (unwired) 9 ("length (rest)")
              (unwired) 9 ("length (rest)")
              (unwired) TRUE ("line mode (F)")
              n2185 = Read from Text File "Read File"(file (use dialog)=w2683, error in=w2684) -> (text=w2651:string)  [unwired: 2 in, 3 out]
              n2186 = local write "String 8"(w2651) -> ()
              n2187 = String Subset(string=w2651, offset (0)=85) -> (substring=w2653:string)  [unwired: 1 in]
              n2188 = String Subset(string=w2651, offset (0)=35, length (rest)=9 ("length (rest)")) -> (substring=w2674:string)
              n2189 = String Subset(string=w2651, offset (0)=55, length (rest)=9 ("length (rest)")) -> (substring=w2659:string)
              n2190 = String Subset(string=w2651, offset (0)=25) -> (substring=w2655:string)  [unwired: 1 in]
              n2191 = String Subset(string=w2651, offset (0)=15, length (rest)=9 ("length (rest)")) -> (substring=w2680:string)
              n2192 = String Subset(string=w2651, offset (0)=0, length (rest)=14 ("length (rest)")) -> (substring=w2677:string)
              n2193 = String Subset(string=w2651, offset (0)=45, length (rest)=9 ("length (rest)")) -> (substring=w2664:string)
              n2194 = String Subset(string=w2651, offset (0)=65, length (rest)=9 ("length (rest)")) -> (substring=w2670:string)
              n2195 = Fract/Exp String To Number(string=w2653) -> (number=w2650:dbl)  [unwired: 3 in, 1 out]
              n2196 = Fract/Exp String To Number(string=w2674) -> (number=w2672:dbl)  [unwired: 3 in, 1 out]
              n2197 = Fract/Exp String To Number(string=w2659) -> (number=w2657:dbl)  [unwired: 3 in, 1 out]
              n2198 = Fract/Exp String To Number(string=w2655) -> (number=w2654:dbl)  [unwired: 3 in, 1 out]
              n2199 = Fract/Exp String To Number(string=w2680) -> (number=w2671:dbl)  [unwired: 3 in, 1 out]
              n2200 = Fract/Exp String To Number(string=w2677) -> (number=w2673:dbl)  [unwired: 3 in, 1 out]
              n2201 = Fract/Exp String To Number(string=w2664) -> (number=w2661:dbl)  [unwired: 3 in, 1 out]
              n2202 = Fract/Exp String To Number(string=w2670) -> (number=w2667:dbl)  [unwired: 3 in, 1 out]
              n2203 = Add(x=w2667, y=0.0) -> (x+y=w2665:dbl)
            }
            n2204 = String To Path(string=w2510) -> (path=w2608:path)
            n2205 = String To Path(string=w2508) -> (path=w2602:path)
            n2206 = local read "Numeric 11"() -> (w2592:i32)
            n2207 = local read "Numeric 13"() -> (w2594:i32)
            n2208 = Open/Create/Replace File "Open File"(file path (use dialog)=w2608) -> (refnum out=w2606:refnum<file>, error out=w2605:errorcluster)  [unwired: 5 in, 1 out]
            n2209 = Open/Create/Replace File "Open File"(file path (use dialog)=w2602) -> (refnum out=w2601:refnum<file>, error out=w2600:errorcluster)  [unwired: 5 in, 1 out]
            n2210 = for {
              N: w2592 -> [_]
              tunnel: w2606 -> [w2721]
              tunnel: w2605 -> [w2720]
              tunnel: [w2710] -> w2572 mode=indexing
              tunnel: [w2708] -> w2570 mode=indexing
              tunnel: [w2709] -> w2565 mode=indexing
              tunnel: w2591 -> [_]
              tunnel: [w2702] -> w2567 mode=indexing
              tunnel: [w2698] -> w2543 mode=indexing
              tunnel: [w2694] -> w2518 mode=indexing
              tunnel: [w2690] -> w2499 mode=indexing
              tunnel: [w2685] -> w2457 mode=indexing
              (unwired) TRUE ("line mode (F)")
              n2211 = Read from Text File "Read File"(file (use dialog)=w2721, error in=w2720) -> (text=w2686:string)  [unwired: 2 in, 3 out]
              n2212 = local write "String 7"(w2686) -> ()
              n2213 = String Subset(string=w2686, offset (0)=85, length (rest)=9 ("length (rest)")) -> (substring=w2689:string)
              n2214 = String Subset(string=w2686, offset (0)=35, length (rest)=9 ("length (rest)")) -> (substring=w2711:string)
              n2215 = String Subset(string=w2686, offset (0)=55, length (rest)=9 ("length (rest)")) -> (substring=w2697:string)
              n2216 = String Subset(string=w2686, offset (0)=25, length (rest)=9 ("length (rest)")) -> (substring=w2691:string)
              n2217 = String Subset(string=w2686, offset (0)=45, length (rest)=9 ("length (rest)")) -> (substring=w2699:string)
              n2218 = String Subset(string=w2686, offset (0)=0, length (rest)=14 ("length (rest)")) -> (substring=w2714:string)
              n2219 = String Subset(string=w2686, offset (0)=15, length (rest)=9 ("length (rest)")) -> (substring=w2717:string)
              n2220 = String Subset(string=w2686, offset (0)=65, length (rest)=9 ("length (rest)")) -> (substring=w2703:string)
              n2221 = Fract/Exp String To Number(string=w2689) -> (number=w2685:dbl)  [unwired: 3 in, 1 out]
              n2222 = Fract/Exp String To Number(string=w2711) -> (number=w2709:dbl)  [unwired: 3 in, 1 out]
              n2223 = Fract/Exp String To Number(string=w2697) -> (number=w2694:dbl)  [unwired: 3 in, 1 out]
              n2224 = Fract/Exp String To Number(string=w2691) -> (number=w2690:dbl)  [unwired: 3 in, 1 out]
              n2225 = Fract/Exp String To Number(string=w2699) -> (number=w2698:dbl)  [unwired: 3 in, 1 out]
              n2226 = Fract/Exp String To Number(string=w2714) -> (number=w2710:dbl)  [unwired: 3 in, 1 out]
              n2227 = Fract/Exp String To Number(string=w2717) -> (number=w2708:dbl)  [unwired: 3 in, 1 out]
              n2228 = Fract/Exp String To Number(string=w2703) -> (number=w2706:dbl)  [unwired: 3 in, 1 out]
              n2229 = Add(x=w2706, y=0.0) -> (x+y=w2702:dbl)
            }
            n2230 = for {
              N: w2594 -> [_]
              tunnel: w2601 -> [w2649]
              tunnel: w2600 -> [w2648]
              tunnel: [w2638] -> w2554 mode=indexing
              tunnel: [w2637] -> w2547 mode=indexing
              tunnel: w2591 -> [_]
              tunnel: [w2626] -> w2552 mode=indexing
              tunnel: [w2631] -> w2549 mode=indexing
              tunnel: [w2627] -> w2539 mode=indexing
              tunnel: [w2622] -> w2514 mode=indexing
              tunnel: [w2618] -> w2495 mode=indexing
              tunnel: [w2613] -> w2455 mode=indexing
              (unwired) 1.0 ("x")
              (unwired) TRUE ("line mode (F)")
              n2231 = Read from Text File "Read File"(file (use dialog)=w2649, error in=w2648) -> (text=w2614:string)  [unwired: 2 in, 3 out]
              n2232 = local write "String 12"(w2614) -> ()
              n2233 = String Subset(string=w2614, offset (0)=85, length (rest)=9 ("length (rest)")) -> (substring=w2616:string)
              n2234 = String Subset(string=w2614, offset (0)=35, length (rest)=9 ("length (rest)")) -> (substring=w2639:string)
              n2235 = String Subset(string=w2614, offset (0)=55, length (rest)=9 ("length (rest)")) -> (substring=w2624:string)
              n2236 = String Subset(string=w2614, offset (0)=25, length (rest)=9 ("length (rest)")) -> (substring=w2620:string)
              n2237 = String Subset(string=w2614, offset (0)=45, length (rest)=9 ("length (rest)")) -> (substring=w2629:string)
              n2238 = String Subset(string=w2614, offset (0)=15, length (rest)=9 ("length (rest)")) -> (substring=w2645:string)
              n2239 = String Subset(string=w2614, offset (0)=0, length (rest)=14 ("length (rest)")) -> (substring=w2642:string)
              n2240 = String Subset(string=w2614, offset (0)=65, length (rest)=9 ("length (rest)")) -> (substring=w2632:string)
              n2241 = Fract/Exp String To Number(string=w2616) -> (number=w2613:dbl)  [unwired: 3 in, 1 out]
              n2242 = Fract/Exp String To Number(string=w2639) -> (number=w2637:dbl)  [unwired: 3 in, 1 out]
              n2243 = Fract/Exp String To Number(string=w2624) -> (number=w2622:dbl)  [unwired: 3 in, 1 out]
              n2244 = Fract/Exp String To Number(string=w2620) -> (number=w2618:dbl)  [unwired: 3 in, 1 out]
              n2245 = Fract/Exp String To Number(string=w2629) -> (number=w2627:dbl)  [unwired: 3 in, 1 out]
              n2246 = Fract/Exp String To Number(string=w2645) -> (number=w2626:dbl)  [unwired: 3 in, 1 out]